vi "Dresden R2R Sputter 03.02.2018 IY24.vi"() -> ()   [LabVIEW 2009] (continued)
                      }
                      n11422 = local read "Semi"() -> (w18198:bool)
                      n11423 = Or(x=w18199, y=w18198) -> (x .or. y?=w18197:bool)
                    }
                  }
                  frame #7 {
                    n11424 = local read "Semi"() -> (w18210:bool)
                    n11425 = case shown="False" w18210 {
                      frame #0 {
                        n11426 = local write "CH1_2trns_12"(TRUE ("CH1_2trns_11")) -> ()
                        n11427 = Wait (ms)(milliseconds to wait=u32 500) -> ()  [unwired: 1 out]
                      }
                      frame #1 {
                      }
                    }
                  }
                }
              }
              frame #1 {
              }
            }
          }
          frame #17 {
            # "CASETTE STOP AND FIX"
            n11428 = local read "Semi"() -> (w18213:bool)
            n11429 = case shown="False" w18213 {
              frame #0 {
                n11430 = stacked-sequence {
                  frame #0 {
                    # "Center Casette stop"
                    n11431 = local read "Semi"() -> (w18214:bool)
                    n11432 = case shown="False" w18214 {
                      frame #0 {
                        n11433 = stacked-sequence {
                          frame #0 {
                            n11434 = while {
                              i -> [w18221]
                              stop <- w18216 stop-if-true
                              n11435 = local read "Ch2_Left_limit_di"() -> (w18215:bool)
                              n11436 = Greater?(x=w18221, y=600) -> (0:w18219:bool)
                              n11437 = case shown="True" w18219 {
                                frame #0 {
                                }
                                frame #1 {
                                n11438 = local write "Semi"(TRUE ("Semi")) -> ()
                                n11439 = local write "Error Message"("Transfer process was cancelled.\nPlease check Casette connections." ("Error Message")) -> ()
                                }
                              }
                              n11440 = case shown="False" w18215 {
                                tunnel: [FALSE TRUE] -> w18218
                                frame #0 {
                                n11441 = Wait Until Next ms Multiple(millisecond multiple=u32 200) -> ()  [unwired: 1 out]
                                }
                                frame #1 {
                                }
                              }
                              n11442 = local read "Semi"() -> (w18217:bool)
                              n11443 = Or(x=w18218, y=w18217) -> (x .or. y?=w18216:bool)
                            }
                          }
                          frame #1 {
                            n11444 = disable-structure shown="Disabled" {
                              frame #0 {
                                n11445 = while {
                                i -> [w18236]
                                stop <- w18231 stop-if-true
                                n11446 = local read "Counter_read_data"() -> (w18228:i16)
                                n11447 = Greater?(x=w18236, y=5000) -> (0:w18234:bool)
                                n11448 = case shown="True" w18234 {
                                frame #0 {
                                }
                                frame #1 {
                                n11449 = local write "Semi"(TRUE ("Semi")) -> ()
                                n11450 = local write "Error Message"("Transfer process was cancelled.\nPlease check Casette connections." ("Error Message")) -> ()
                                }
                                }
                                n11451 = In Range and Coerce(upper limit=i16 2209, x=w18228, lower limit=i16 2199 ("upper limit")) -> (In Range?=w18227:bool)  [unwired: 1 out]
                                n11452 = case shown="True" w18227 {
                                tunnel: [FALSE TRUE] -> w18233
                                frame #0 {
                                }
                                frame #1 {
                                n11453 = Wait Until Next ms Multiple(millisecond multiple=u32 500) -> ()  [unwired: 1 out]
                                }
                                }
                                n11454 = local read "Semi"() -> (w18232:bool)
                                n11455 = Or(x=w18233, y=w18232) -> (x .or. y?=w18231:bool)
                                }
                              }
                              frame #1 {
                              }
                            }
                          }
                          frame #2 {
                            n11456 = while {
                              i -> [w18248]
                              stop <- w18243 stop-if-true
                              n11457 = local read "Casette_servo_start/stop_di"() -> (w18242:bool)
                              n11458 = Greater?(x=w18248, y=50) -> (0:w18246:bool)
                              n11459 = case shown="True" w18246 {
                                frame #0 {
                                }
                                frame #1 {
                                n11460 = local write "Semi"(TRUE ("Semi")) -> ()
                                n11461 = local write "Error Message"("Transfer process was cancelled.\nPlease check Casette connections." ("Error Message")) -> ()
                                }
                              }
                              n11462 = case shown="True" w18242 {
                                tunnel: [TRUE FALSE] -> w18245
                                frame #0 {
                                }
                                frame #1 {
                                n11463 = Wait Until Next ms Multiple(millisecond multiple=u32 200) -> ()  [unwired: 1 out]
                                n11464 = local write "Casette_servo_start/stop_do"(FALSE ("Casette_servo_start/stop_di")) -> ()
                                }
                              }
                              n11465 = local read "Semi"() -> (w18244:bool)
                              n11466 = Or(x=w18245, y=w18244) -> (x .or. y?=w18243:bool)
                            }
                          }
                          frame #3 {
                            n11467 = local read "Semi"() -> (w18255:bool)
                            n11468 = case shown="False" w18255 {
                              frame #0 {
                                n11469 = Wait (ms)(milliseconds to wait=u32 200) -> ()  [unwired: 1 out]
                              }
                              frame #1 {
                              }
                            }
                          }
                          frame #4 {
                            n11470 = local read "Semi"() -> (w18257:bool)
                            n11471 = case shown="False" w18257 {
                              frame #0 {
                                n11472 = local write "Cassette_servo_speed_value"(u16 0 ("Cassette_servo_speed_value")) -> ()
                              }
                              frame #1 {
                              }
                            }
                          }
                          frame #5 {
                            n11473 = local read "Semi"() -> (w18259:bool)
                            n11474 = case shown="False" w18259 {
                              frame #0 {
                                n11475 = Wait (ms)(milliseconds to wait=u32 200) -> ()  [unwired: 1 out]
                              }
                              frame #1 {
                              }
                            }
                          }
                          frame #6 {
                            n11476 = local read "Semi"() -> (w18261:bool)
                            n11477 = case shown="False" w18261 {
                              frame #0 {
                                n11478 = local write "Cassette_servo_speed_auto_set"(TRUE ("Cassette_servo_speed_auto_set")) -> ()
                              }
                              frame #1 {
                              }
                            }
                          }
                          frame #7 {
                            n11479 = local read "Semi"() -> (w18263:bool)
                            n11480 = case shown="False" w18263 {
                              frame #0 {
                                n11481 = Wait (ms)(milliseconds to wait=u32 200) -> ()  [unwired: 1 out]
                              }
                              frame #1 {
                              }
                            }
                          }
                          frame #8 {
                            n11482 = local read "Semi"() -> (w18265:bool)
                            n11483 = case shown="False" w18265 {
                              frame #0 {
                                n11484 = local write "CH1_2trns_13"(TRUE ("CH1_2trns_9")) -> ()
                                n11485 = Wait (ms)(milliseconds to wait=u32 500) -> ()  [unwired: 1 out]
                              }
                              frame #1 {
                              }
                            }
                          }
                        }
                      }
                      frame #1 {
                      }
                    }
                  }
                  frame #1 {
                    # "CASETTE FIX DOWN CH2"
                    n11486 = local read "Semi"() -> (w18268:bool)
                    n11487 = case shown="False" w18268 {
                      frame #0 {
                        n11488 = stacked-sequence {
                          frame #0 {
                            n11489 = local read "Semi"() -> (w18269:bool)
                            n11490 = case shown="False" w18269 {
                              frame #0 {
                                n11491 = while {
                                i -> [w18276]
                                stop <- w18271 stop-if-true
                                n11492 = Greater?(x=w18276, y=50) -> (0:w18274:bool)
                                n11493 = local read "Ch2_Cst_fix_down_di"() -> (w18270:bool)
                                n11494 = case shown="True" w18274 {
                                frame #0 {
                                }
                                frame #1 {
                                n11495 = local write "Semi"(TRUE ("Semi")) -> ()
                                n11496 = local write "Error Message"("Up/Down positions could not reach\nthe down position.\nPlease check connections." ("Error Message")) -> ()
                                }
                                }
                                n11497 = case shown="False" w18270 {
                                tunnel: [FALSE TRUE] -> w18273
                                frame #0 {
                                n11498 = Wait Until Next ms Multiple(millisecond multiple=u32 200) -> ()  [unwired: 1 out]
                                n11499 = local write "Ch2_Cst_fix_do"(TRUE ("Ch1_pet_cool_up_do")) -> ()
                                }
                                frame #1 {
                                }
                                }
                                n11500 = local read "Semi"() -> (w18272:bool)
                                n11501 = Or(x=w18273, y=w18272) -> (x .or. y?=w18271:bool)
                                }
                              }
                              frame #1 {
                              }
                            }
                          }
                          frame #1 {
                            n11502 = local read "Semi"() -> (w18283:bool)
                            n11503 = case shown="False" w18283 {
                              frame #0 {
                                n11504 = local write "CH1_2trns_14"(TRUE ("CH1_2trns_9")) -> ()
                                n11505 = Wait (ms)(milliseconds to wait=u32 500) -> ()  [unwired: 1 out]
                              }
                              frame #1 {
                              }
                            }
                          }
                        }
                      }
                      frame #1 {
                      }
                    }
                  }
                  frame #2 {
                    n11506 = local read "Semi"() -> (w18286:bool)
                    n11507 = case shown="False" w18286 {
                      frame #0 {
                        n11508 = stacked-sequence {
                          frame #0 {
                            n11509 = local read "Semi"() -> (w18287:bool)
                            n11510 = case shown="False" w18287 {
                              frame #0 {
                                n11511 = while {
                                i -> [w18294]
                                stop <- w18289 stop-if-true
                                n11512 = Greater?(x=w18294, y=50) -> (0:w18292:bool)
                                n11513 = local read "Ch1_Trns_gv_bp2_di"() -> (w18288:bool)
                                n11514 = case shown="True" w18292 {
                                frame #0 {
                                }
                                frame #1 {
                                n11515 = local write "Semi"(TRUE ("Semi")) -> ()
                                n11516 = local write "Error Message"("Transfer process was cancelled.\nPlease check CH1-Trns-GV connections." ("Error Message")) -> ()
                                }
                                }
                                n11517 = case shown="True" w18288 {
                                tunnel: [TRUE FALSE] -> w18291
                                frame #0 {
                                }
                                frame #1 {
                                n11518 = Wait Until Next ms Multiple(millisecond multiple=u32 200) -> ()  [unwired: 1 out]
                                n11519 = local write "Ch1_Trns_gv_bp2_do"(FALSE ("Ch1_pet_cool_up_do")) -> ()
                                }
                                }
                                n11520 = local read "Semi"() -> (w18290:bool)
                                n11521 = Or(x=w18291, y=w18290) -> (x .or. y?=w18289:bool)
                                }
                              }
                              frame #1 {
                              }
                            }
                          }
                          frame #1 {
                            n11522 = local read "Semi"() -> (w18301:bool)
                            n11523 = case shown="False" w18301 {
                              frame #0 {
                                n11524 = Wait (ms)(milliseconds to wait=u32 500) -> ()  [unwired: 1 out]
                              }
                              frame #1 {
                              }
                            }
                          }
                          frame #2 {
                            n11525 = local read "Semi"() -> (w18303:bool)
                            n11526 = case shown="False" w18303 {
                              frame #0 {
                                n11527 = while {
                                i -> [w18310]
                                stop <- w18305 stop-if-true
                                n11528 = Greater?(x=w18310, y=50) -> (0:w18308:bool)
                                n11529 = local read "Ch2_trns_gv_bp_di"() -> (w18304:bool)
                                n11530 = case shown="True" w18308 {
                                frame #0 {
                                }
                                frame #1 {
                                n11531 = local write "Semi"(TRUE ("Semi")) -> ()
                                n11532 = local write "Error Message"("Transfer process was cancelled.\nPlease check CH1-Trns-GV connections." ("Error Message")) -> ()
                                }
                                }
                                n11533 = case shown="True" w18304 {
                                tunnel: [TRUE FALSE] -> w18307
                                frame #0 {
                                }
                                frame #1 {
                                n11534 = Wait Until Next ms Multiple(millisecond multiple=u32 200) -> ()  [unwired: 1 out]
                                n11535 = local write "Ch2_trns_gv_bp_do"(FALSE ("Ch1_pet_cool_up_do")) -> ()
                                }
                                }
                                n11536 = local read "Semi"() -> (w18306:bool)
                                n11537 = Or(x=w18307, y=w18306) -> (x .or. y?=w18305:bool)
                                }
                              }
                              frame #1 {
                              }
                            }
                          }
                          frame #3 {
                            n11538 = local read "Semi"() -> (w18317:bool)
                            n11539 = case shown="False" w18317 {
                              frame #0 {
                                n11540 = Wait (ms)(milliseconds to wait=u32 500) -> ()  [unwired: 1 out]
                              }
                              frame #1 {
                              }
                            }
                          }
                        }
                      }
                      frame #1 {
                      }
                    }
                  }
                  frame #3 {
                    n11541 = local read "Semi"() -> (w18319:bool)
                    n11542 = case shown="False" w18319 {
                      frame #0 {
                        n11543 = stacked-sequence {
                          frame #0 {
                            n11544 = local read "Semi"() -> (w18320:bool)
                            n11545 = case shown="False" w18320 {
                              frame #0 {
                                n11546 = local write "Ch1_Trns_gv_open_do"(FALSE ("Ch1_pet_cool_up_do")) -> ()
                              }
                              frame #1 {
                              }
                            }
                          }
                          frame #1 {
                            n11547 = local read "Semi"() -> (w18322:bool)
                            n11548 = case shown="False" w18322 {
                              frame #0 {
                                n11549 = while {
                                i -> [w18329]
                                stop <- w18324 stop-if-true
                                n11550 = Greater?(x=w18329, y=500) -> (0:w18327:bool)
                                n11551 = local read "Ch1_Trns_gv_close_di"() -> (w18323:bool)
                                n11552 = case shown="True" w18327 {
                                frame #0 {
                                }
                                frame #1 {
                                n11553 = local write "Semi"(TRUE ("Semi")) -> ()
                                n11554 = local write "Error Message"("Transfer process was cancelled.\nPlease check  GV connections." ("Error Message")) -> ()
                                }
                                }
                                n11555 = case shown="False" w18323 {
                                tunnel: [FALSE TRUE] -> w18326
                                frame #0 {
                                n11556 = Wait Until Next ms Multiple(millisecond multiple=u32 200) -> ()  [unwired: 1 out]
                                n11557 = local write "Ch1_Trns_gv_close_do"(TRUE ("Ch1_pet_cool_up_do")) -> ()
                                }
                                frame #1 {
                                }
                                }
                                n11558 = local read "Semi"() -> (w18325:bool)
                                n11559 = Or(x=w18326, y=w18325) -> (x .or. y?=w18324:bool)
                                }
                              }
                              frame #1 {
                              }
                            }
                          }
                          frame #2 {
                            n11560 = local read "Semi"() -> (w18336:bool)
                            n11561 = case shown="False" w18336 {
                              frame #0 {
                                n11562 = local write "CH1_2trns_17"(TRUE ("CH1_2trns_9")) -> ()
                                n11563 = Wait (ms)(milliseconds to wait=u32 500) -> ()  [unwired: 1 out]
                              }
                              frame #1 {
                              }
                            }
                          }
                        }
                      }
                      frame #1 {
                      }
                    }
                  }
                  frame #4 {
                    # "PET COOL DOWN OF CH2"
                    n11564 = local read "Semi"() -> (w18339:bool)
                    n11565 = case shown="False" w18339 {
                      frame #0 {
                        n11566 = stacked-sequence {
                          frame #0 {
                            n11567 = local read "Semi"() -> (w18340:bool)
                            n11568 = case shown="False" w18340 {
                              frame #0 {
                                n11569 = local write "Ch2_Pet_cool_up_do"(FALSE ("Ch1_pet_cool_up_do")) -> ()
                              }
                              frame #1 {
                              }
                            }
                          }
                          frame #1 {
                            n11570 = local read "Semi"() -> (w18342:bool)
                            n11571 = case shown="False" w18342 {
                              frame #0 {
                                n11572 = while {
                                i -> [w18349]
                                stop <- w18344 stop-if-true
                                n11573 = Greater?(x=w18349, y=300) -> (0:w18347:bool)
                                n11574 = case shown="True" w18347 {
                                frame #0 {
                                }
                                frame #1 {
                                n11575 = local write "Semi"(TRUE ("Semi")) -> ()
                                n11576 = local write "Error Message"("SBS Cool Up/Down positions could not reach\nthe down position.\nPlease check connections." ("Error Message")) -> ()
                                }
                                }
                                n11577 = local read "Ch2_Pet_cool_down_di"() -> (w18343:bool)
                                n11578 = case shown="False" w18343 {
                                tunnel: [FALSE TRUE] -> w18346
                                frame #0 {
                                n11579 = Wait Until Next ms Multiple(millisecond multiple=u32 200) -> ()  [unwired: 1 out]
                                n11580 = local write "Ch2_Pet_cool_down_do"(TRUE ("Ch1_pet_cool_up_do")) -> ()
                                }
                                frame #1 {
                                }
                                }
                                n11581 = local read "Semi"() -> (w18345:bool)
                                n11582 = Or(x=w18346, y=w18345) -> (x .or. y?=w18344:bool)
                                }
                              }
                              frame #1 {
                              }
                            }
                          }
                          frame #2 {
                            n11583 = local read "Semi"() -> (w18356:bool)
                            n11584 = case shown="False" w18356 {
                              frame #0 {
                                n11585 = local write "CH1_2trns_15"(TRUE ("CH1_2trns_9")) -> ()
                                n11586 = Wait (ms)(milliseconds to wait=u32 500) -> ()  [unwired: 1 out]
                              }
                              frame #1 {
                              }
                            }
                          }
                        }
                      }
                      frame #1 {
                      }
                    }
                  }
                  frame #5 {
                    # "SRV PIS FOR"
                    n11587 = local read "Semi"() -> (w18359:bool)
                    n11588 = case shown="False" w18359 {
                      frame #0 {
                        n11589 = stacked-sequence {
                          frame #0 {
                            n11590 = local read "Semi"() -> (w18360:bool)
                            n11591 = case shown="False" w18360 {
                              frame #0 {
                                n11592 = local write "Ch2_SRV1_PIST_Back_do"(FALSE ("Ch1_pet_cool_up_do")) -> ()
                              }
                              frame #1 {
                              }
                            }
                          }
                          frame #1 {
                            n11593 = local read "Semi"() -> (w18362:bool)
                            n11594 = case shown="False" w18362 {
                              frame #0 {
                                n11595 = while {
                                i -> [w18369]
                                stop <- w18364 stop-if-true
                                n11596 = Greater?(x=w18369, y=100) -> (0:w18367:bool)
                                n11597 = local read "Ch2_SRV1_PIST For_di"() -> (w18363:bool)
                                n11598 = case shown="True" w18367 {
                                frame #0 {
                                }
                                frame #1 {
                                n11599 = local write "Semi"(TRUE ("Semi")) -> ()
                                n11600 = local write "Error Message"("For/Back positions could not reach\nthe forward position.\nPlease check connections." ("Error Message")) -> ()
                                }
                                }
                                n11601 = case shown="False" w18363 {
                                tunnel: [FALSE TRUE] -> w18366
                                frame #0 {
                                n11602 = Wait Until Next ms Multiple(millisecond multiple=u32 200) -> ()  [unwired: 1 out]
                                n11603 = local write "Ch2_SRV1_PIST For_do"(TRUE ("Ch1_pet_cool_up_do")) -> ()
                                }
                                frame #1 {
                                }
                                }
                                n11604 = local read "Semi"() -> (w18365:bool)
                                n11605 = Or(x=w18366, y=w18365) -> (x .or. y?=w18364:bool)
                                }
                              }
                              frame #1 {
                              }
                            }
                          }
                          frame #2 {
                            n11606 = local read "Semi"() -> (w18376:bool)
                            n11607 = case shown="False" w18376 {
                              frame #0 {
                                n11608 = local write "CH1_2trns_16"(TRUE ("CH1_2trns_9")) -> ()
                                n11609 = Wait (ms)(milliseconds to wait=u32 500) -> ()  [unwired: 1 out]
                              }
                              frame #1 {
                              }
                            }
                          }
                        }
                      }
                      frame #1 {
                      }
                    }
                  }
                }
              }
              frame #1 {
              }
            }
          }
          frame #18 {
            # "Sensors deactive"
            n11610 = local read "Semi"() -> (w18379:bool)
            n11611 = case shown="False" w18379 {
              frame #0 {
                n11612 = stacked-sequence {
                  frame #0 {
                    n11613 = local read "Semi"() -> (w18380:bool)
                    n11614 = case shown="False" w18380 {
                      frame #0 {
                        n11615 = while {
                          i -> [w18383]
                          stop <- w18384 stop-if-true
                          n11616 = Greater?(x=w18383, y=50) -> (0:w18381:bool)
                          n11617 = local read "Cnt_Right_slow_di"() -> (w18387:bool)
                          n11618 = case shown="True" w18381 {
                            frame #0 {
                            }
                            frame #1 {
                              n11619 = local write "Semi"(TRUE ("Semi")) -> ()
                              n11620 = local write "Error Message"("Transfer process was\ncancelled.Please check right slow sensor." ("Error Message")) -> ()
                            }
                          }
                          n11621 = case shown="False" w18387 {
                            tunnel: [FALSE ("Ch1_pet_cool_up_do") TRUE ("Ch1_pet_cool_up_do")] -> w18386
                            frame #0 {
                              n11622 = Wait Until Next ms Multiple(millisecond multiple=u32 200) -> ()  [unwired: 1 out]
                              n11623 = local write "Cnt_Right_slow_do"(TRUE ("Ch1_pet_cool_up_do")) -> ()
                            }
                            frame #1 {
                            }
                          }
                          n11624 = local read "Semi"() -> (w18385:bool)
                          n11625 = Or(x=w18386, y=w18385) -> (x .or. y?=w18384:bool)
                        }
                      }
                      frame #1 {
                      }
                    }
                  }
                  frame #1 {
                    n11626 = local read "Semi"() -> (w18394:bool)
                    n11627 = case shown="False" w18394 {
                      frame #0 {
                        n11628 = while {
                          i -> [w18397]
                          stop <- w18398 stop-if-true
                          n11629 = Greater?(x=w18397, y=50) -> (0:w18395:bool)
                          n11630 = local read "Cnt_Right_limit_di"() -> (w18401:bool)
                          n11631 = case shown="True" w18395 {
                            frame #0 {
                            }
                            frame #1 {
                              n11632 = local write "Semi"(TRUE ("Semi")) -> ()
                              n11633 = local write "Error Message"("Transfer process was\ncancelled.Please check right limit sensor." ("Error Message")) -> ()
                            }
                          }
                          n11634 = case shown="False" w18401 {
                            tunnel: [FALSE ("Ch1_pet_cool_up_do") TRUE ("Ch1_pet_cool_up_do")] -> w18400
                            frame #0 {
                              n11635 = Wait Until Next ms Multiple(millisecond multiple=u32 200) -> ()  [unwired: 1 out]
                              n11636 = local write "Cnt_Right_limit_do"(TRUE ("Ch1_pet_cool_up_do")) -> ()
                            }
                            frame #1 {
                            }
                          }
                          n11637 = local read "Semi"() -> (w18399:bool)
                          n11638 = Or(x=w18400, y=w18399) -> (x .or. y?=w18398:bool)
                        }
                      }
                      frame #1 {
                      }
                    }
                  }
                  frame #2 {
                    n11639 = local read "Semi"() -> (w18408:bool)
                    n11640 = case shown="False" w18408 {
                      frame #0 {
                        n11641 = while {
                          i -> [w18411]
                          stop <- w18412 stop-if-true
                          n11642 = Greater?(x=w18411, y=50) -> (0:w18409:bool)
                          n11643 = local read "Cnt_Left_slow_di"() -> (w18415:bool)
                          n11644 = case shown="True" w18409 {
                            frame #0 {
                            }
                            frame #1 {
                              n11645 = local write "Semi"(TRUE ("Semi")) -> ()
                              n11646 = local write "Error Message"("Transfer process was\ncancelled.Please check left slow sensor." ("Error Message")) -> ()
                            }
                          }
                          n11647 = case shown="False" w18415 {
                            tunnel: [FALSE ("Ch1_pet_cool_up_do") TRUE ("Ch1_pet_cool_up_do")] -> w18414
                            frame #0 {
                              n11648 = Wait Until Next ms Multiple(millisecond multiple=u32 200) -> ()  [unwired: 1 out]
                              n11649 = local write "Cnt_Left_slow_do"(TRUE ("Ch1_pet_cool_up_do")) -> ()
                            }
                            frame #1 {
                            }
                          }
                          n11650 = local read "Semi"() -> (w18413:bool)
                          n11651 = Or(x=w18414, y=w18413) -> (x .or. y?=w18412:bool)
                        }
                      }
                      frame #1 {
                      }
                    }
                  }
                  frame #3 {
                    n11652 = local read "Semi"() -> (w18422:bool)
                    n11653 = case shown="False" w18422 {
                      frame #0 {
                        n11654 = while {
                          i -> [w18425]
                          stop <- w18426 stop-if-true
                          n11655 = Greater?(x=w18425, y=50) -> (0:w18423:bool)
                          n11656 = local read "Cnt_Left_limit_di"() -> (w18429:bool)
                          n11657 = case shown="True" w18423 {
                            frame #0 {
                            }
                            frame #1 {
                              n11658 = local write "Semi"(TRUE ("Semi")) -> ()
                              n11659 = local write "Error Message"("Transfer process was\ncancelled.Please check left limit sensor." ("Error Message")) -> ()
                            }
                          }
                          n11660 = case shown="False" w18429 {
                            tunnel: [FALSE ("Ch1_pet_cool_up_do") TRUE ("Ch1_pet_cool_up_do")] -> w18428
                            frame #0 {
                              n11661 = Wait Until Next ms Multiple(millisecond multiple=u32 200) -> ()  [unwired: 1 out]
                              n11662 = local write "Cnt_Left_limit_do"(TRUE ("Ch1_pet_cool_up_do")) -> ()
                            }
                            frame #1 {
                            }
                          }
                          n11663 = local read "Semi"() -> (w18427:bool)
                          n11664 = Or(x=w18428, y=w18427) -> (x .or. y?=w18426:bool)
                        }
                      }
                      frame #1 {
                      }
                    }
                  }
                  frame #4 {
                    n11665 = local read "Semi"() -> (w18436:bool)
                    n11666 = case shown="False" w18436 {
                      frame #0 {
                        n11667 = local write "CH1_2trns_18"(TRUE ("CH1_2trns_7")) -> ()
                        n11668 = Wait (ms)(milliseconds to wait=u32 500) -> ()  [unwired: 1 out]
                      }
                      frame #1 {
                      }
                    }
                  }
                }
              }
              frame #1 {
              }
            }
          }
          frame #19 {
            n11669 = local read "Semi"() -> (w18439:bool)
            n11670 = case shown="False" w18439 {
              frame #0 {
                n11671 = local write "CH1_2trns_19"(TRUE ("CH1_2trns_18")) -> ()
                n11672 = local write "Cnt_Do_Buzzer"(TRUE ("Transfer_ch1_2")) -> ()
                n11673 = Wait (ms)(milliseconds to wait=u32 1500) -> ()  [unwired: 1 out]
              }
              frame #1 {
              }
            }
          }
          frame #20 {
            n11674 = local read "Semi"() -> (w18443:bool)
            n11675 = case shown="False" w18443 {
              frame #0 {
                n11676 = local write "ch_present_position"(2.0 ("ch_present_position")) -> ()
                n11677 = local write "Transfer_ch1_2"(FALSE ("Transfer_ch1_2")) -> ()
                n11678 = local write "Cnt_Do_Buzzer"(FALSE ("Transfer_ch1_2")) -> ()
                n11679 = Wait (ms)(milliseconds to wait=u32 500) -> ()  [unwired: 1 out]
              }
              frame #1 {
              }
            }
          }
        }
      }
      frame #2 {
        n11680 = stacked-sequence {
          frame #0 {
            n11681 = Wait (ms)(milliseconds to wait=u32 1500) -> ()  [unwired: 1 out]
            n11682 = local write "Clean_trnsfr_2_1"(TRUE ("Clean_trnsfr_1_2")) -> ()
            n11683 = local write "system_status"("Chamber 2 to Chamber 1 Transfer Process in Progress." ("system_status")) -> ()
            n11684 = local write "final_process_messages"("Chamber 2 to Chamber 1  Transfer Process was completed." ("final_process_messages")) -> ()
          }
          frame #1 {
            n11685 = stacked-sequence {
              frame #0 {
                n11686 = local write "Routine_check_transfer"(TRUE ("Routine_check_transfer")) -> ()
                n11687 = Wait (ms)(milliseconds to wait=u32 100) -> ()  [unwired: 1 out]
              }
              frame #1 {
                n11688 = while {
                  i -> [w18461]
                  stop <- w18457 stop-if-true
                  n11689 = Greater Or Equal?(x=w18461, y=1500) -> (x >= y?=w18458:bool)
                  n11690 = Wait Until Next ms Multiple(millisecond multiple=u32 200) -> ()  [unwired: 1 out]
                  n11691 = case shown="True" w18458 {
                    frame #0 {
                    }
                    frame #1 {
                      # "Hata mesajı"
                      n11692 = local write "Semi"(TRUE ("Semi")) -> ()
                    }
                  }
                  n11693 = local read "Routine_check_transfer"() -> (w18454:bool)
                  n11694 = local read "Semi"() -> (w18456:bool)
                  n11695 = Not(x=w18454) -> (.not. x?=w18455:bool)
                  n11696 = Or(x=w18455, y=w18456) -> (x .or. y?=w18457:bool)
                }
              }
              frame #2 {
                n11697 = Wait (ms)(milliseconds to wait=u32 500) -> ()  [unwired: 1 out]
              }
            }
          }
          frame #2 {
            # "STARTED UP CH1"
            n11698 = disable-structure shown="Disabled" {
              frame #0 {
                n11699 = local read "Semi"() -> (w18464:bool)
                n11700 = case shown="False" w18464 {
                  frame #0 {
                    n11701 = local read "started_up_ch1"() -> (w18465:bool)
                    n11702 = case shown="False" w18465 {
                      frame #0 {
                        n11703 = stacked-sequence {
                          frame #0 {
                            n11704 = local read "Semi"() -> (w18466:bool)
                            n11705 = case shown="False" w18466 {
                              frame #0 {
                                n11706 = local write "Start_up_ch1"(TRUE ("Start_up_ch2")) -> ()
                              }
                              frame #1 {
                              }
                            }
                          }
                          frame #1 {
                            n11707 = local read "Semi"() -> (w18468:bool)
                            n11708 = case shown="False" w18468 {
                              frame #0 {
                                n11709 = Wait (ms)(milliseconds to wait=u32 16000) -> ()  [unwired: 1 out]
                              }
                              frame #1 {
                              }
                            }
                          }
                          frame #2 {
                            n11710 = local read "Semi"() -> (w18470:bool)
                            n11711 = case shown="False" w18470 {
                              frame #0 {
                                n11712 = while {
                                i -> [w18475]
                                stop <- w18472 stop-if-true
                                n11713 = Greater?(x=w18475, y=80) -> (0:w18473:bool)
                                n11714 = local read "started_up_ch1"() -> (w18471:bool)
                                n11715 = case shown="True" w18473 {
                                frame #0 {
                                }
                                frame #1 {
                                n11716 = local write "Semi"(TRUE ("Semi")) -> ()
                                n11717 = local write "Error Message"("Chamber 1 Pressure is not suitable  \nfor transfer process!\nPlease check connections." ("Error Message")) -> ()
                                }
                                }
                                n11718 = case shown="False" w18471 {
                                tunnel: [FALSE TRUE] -> w18472
                                frame #0 {
                                n11719 = Wait Until Next ms Multiple(millisecond multiple=u32 200) -> ()  [unwired: 1 out]
                                }
                                frame #1 {
                                }
                                }
                                }
                              }
                              frame #1 {
                              }
                            }
                          }
                          frame #3 {
                            n11720 = local read "Semi"() -> (w18481:bool)
                            n11721 = case shown="False" w18481 {
                              frame #0 {
                                n11722 = local write "CH1_2_trns_0"(TRUE ("CH1_2_trns_0")) -> ()
                                n11723 = Wait (ms)(milliseconds to wait=u32 1000) -> ()  [unwired: 1 out]
                              }
                              frame #1 {
                              }
                            }
                          }
                        }
                      }
                      frame #1 {
                      }
                    }
                  }
                  frame #1 {
                  }
                }
              }
              frame #1 {
              }
            }
          }
          frame #3 {
            # "STARTED UP CH2"
            n11724 = disable-structure shown="Disabled" {
              frame #0 {
                n11725 = local read "Semi"() -> (w18484:bool)
                n11726 = case shown="False" w18484 {
                  frame #0 {
                    n11727 = local read "started_up_ch2"() -> (w18485:bool)
                    n11728 = case shown="False" w18485 {
                      frame #0 {
                        n11729 = stacked-sequence {
                          frame #0 {
                            n11730 = local read "Semi"() -> (w18486:bool)
                            n11731 = case shown="False" w18486 {
                              frame #0 {
                                n11732 = local write "Start_up_ch2"(TRUE ("Start_up_ch2")) -> ()
                              }
                              frame #1 {
                              }
                            }
                          }
                          frame #1 {
                            n11733 = local read "Semi"() -> (w18488:bool)
                            n11734 = case shown="False" w18488 {
                              frame #0 {
                                n11735 = Wait (ms)(milliseconds to wait=u32 18000) -> ()  [unwired: 1 out]
                              }
                              frame #1 {
                              }
                            }
                          }